vi "UHR-Fleezers Control (host) - 10.7.vi"() -> ()   [LabVIEW 2010] (continued)
    "T2 X" <- w1093
    n789 = Absolute Value(x=w1115) -> (abs(x)=w1116:dbl[])
    n790 = Absolute Value(x=w1114) -> (abs(x)=w1117:dbl[])
    n791 = call <vilib>:"Mean.vi"("X"=w1115) -> ("mean"=w1094:dbl)  [unwired: 1 out]
    "T1 X" <- w1094
    n792 = Add(x=w1116, y=w1117) -> (x+y=w1118:dbl[])
    n793 = Bundle By Name(cluster=w1150, "Y"=w1112) -> (w1080:waveform(dbl))
    "Bead Separation" <- w1080
    n794 = Divide(x=w1118, y=2.0) -> (x/y=→"Vec Mean of T1 T2":dbl[])
    n795 = case shown="True" w1127 {
      tunnel: w1169 -> [_ w2031]
      tunnel: w1168 -> [_ w2030]
      tunnel: w1167 -> [_ w2029]
      tunnel: w1164 -> [_ w2028]
      tunnel: w1089 -> [_ w2027]
      frame False {
      }
      frame True {
        n796 = property on="Force" class="WFChart (strict)"("YScale.NameLbl.Text"=w2031) -> ()  [unwired: 2 in, 2 out]
        n797 = property on="T2 X" class="DigNum (strict)"("Caption.Text"=w2029) -> ()  [unwired: 2 in, 2 out]
        n798 = property on="T1 X" class="DigNum (strict)"("Caption.Text"=w2030) -> ()  [unwired: 2 in, 2 out]
        n799 = property on="Mean" class="DigNum (strict)"("Caption.Text"=w2028) -> ()  [unwired: 2 in, 2 out]
        n800 = property on="Difference" class="DigNum (strict)"("Caption.Text"=w2027) -> ()  [unwired: 2 in, 2 out]
      }
    }
    n801 = local read "Tether"() -> (w1121:bool)
    n802 = Absolute Value(x=w1094) -> (abs(x)=w1091:dbl)
    n803 = Absolute Value(x=w1093) -> (abs(x)=w1090:dbl)
    n804 = Add(x=w1091, y=w1090) -> (x+y=w1166:dbl)
    n805 = Subtract(x=w1091, y=w1090) -> (x-y=→"Difference":dbl)
    n806 = feedback #18(w1112) -> (w1111:dbl[])
    n807 = Divide(x=w1166, y=2.0) -> (x/y=w1120:dbl)
    "Mean" <- w1120
    n808 = case shown="True" w1121 {
      tunnel: w1120 -> [_ w1572]
      frame False {
      }
      frame True {
        n809 = Greater?(x="Lost Tether Alarm Threshold (pN)", y=w1572) -> (0:w1570:bool)
        n810 = case shown="True" w1570 {
          frame False {
          }
          frame True {
            n811 = flat-sequence {
              frame #0 {
                # "stop only if saving"
                n812 = local read "Saving..."() -> (w1585:bool)
                n813 = And(x=w1585, y="TA Cancel Save?") -> (x .and. y?=w1584:bool)
                n814 = local write "Stop Saving"(w1584) -> ()
              }
              frame #1 {
                n815 = case shown="True" "TA Green Off?" {
                  frame False {
                  }
                  frame True {
                    w1588 = FALSE ("Fl. Triggered...")
                    n816 = local write "Fl. Triggered..."(w1588) -> ()
                    n817 = property on="Green Laser ON/Interlacing" class="Bool (strict)"("Val(Sgnl)"=w1588) -> ()  [unwired: 2 in, 2 out]
                  }
                }
              }
            }
            n818 = local read "Time tether formed"() -> (w1579:timestamp)
            n819 = Get Date/Time In Seconds() -> (seconds since 1Jan1904=w1580:timestamp)
            n820 = Subtract(x=w1580, y=w1579) -> (x-y=w1578:dbl)
            n821 = Number To Decimal String(number=w1578) -> (decimal integer string=w1575:string)  [unwired: 1 out]
            n822 = local read "Messages"() -> (w1582:string)
            n823 = call <vilib>:"Beep.vi"() -> ()  [unwired: 3 in, 9 out]
            n824 = Concatenate Strings("Lost tether (" ("Message to add"), w1575, " s)." ("string")) -> (w1577:string)
            n825 = local write "Tether"(FALSE ("Tether")) -> ()
            n826 = call "Update messages.vi"("Message to add"=w1577, "Old message string"=w1582) -> ("New message string"=w1581:string)
            n827 = local write "Messages"(w1581) -> ()
            n828 = property on="Trap Pos. FB ON" class="Bool (strict)"("Val(Sgnl)"=FALSE ("Value (Signaling)")) -> ()  [unwired: 2 in, 2 out]
          }
        }
      }
    }
    n829 = Build Array (concatenate)(w1112, w1111) -> (w1110:dbl[])
    n830 = Split 1D Array(array=w1110, index=w992) -> (first subarray=w1106:dbl[])  [unwired: 1 out]
    n831 = feedback-in #18(w1106) -> ()
    n832 = call <vilib>:"Mean.vi"("X"=w1106) -> ("mean"=w1105:dbl)  [unwired: 1 out]
    "Bead Mean (nm)" <- w1105
    n833 = Subtract(x=w1106, y=w1105) -> (x-y=w1104:dbl[])
    n834 = Square(x=w1104) -> (x^2=w1103:dbl[])
    n835 = call <vilib>:"Mean.vi"("X"=w1103) -> ("mean"=w1102:dbl)  [unwired: 1 out]
    n836 = Square Root(x=w1102) -> (sqrt(x)=w1101:dbl)
    n837 = Multiply(x=10.0, y=w1101) -> (x*y=→"RMS (Ang)":dbl)
    n838 = xnode "Read/Write Control"("FPGA VI Reference In"=w1142, "error in"=w1141) -> ("FPGA VI Reference Out"=w1260:T19, "error out"=w1254:errorcluster, "AI2 Y Sum Set 1"=w1250:i16, "AI2 Y Sum Set 2"=w1249:i16, "AI1 X Set 1"=w1026:fxp<+/-,16,1>, "AI1 X Set 2"=w1025:fxp<+/-,16,1>, "Trap Pos FB Int Signal"=→"Trap Pos FB Int Signal":fxp<+/-,24,9>, "Trap Pos FB Int-Norm Signal"=→"Trap Pos FB Int-Norm Signal":fxp<+/-,16,1>, "Trap Pos FB Action"=w1019:i64, "Scanning"=→"AOD Scanning":bool, "Scan I"=→"AOD Scan I":u64, "Scanning MCL"=w1252:bool, "Scan I (MCL)"=→"MCL Scan I":u64, "Green FB Signals"=w1189:T38)  [unwired: 1 out]
    "MCL Scanning" <- w1252
    "Trap Pos FB Action" <- w1019
    n839 = local read "AI2 (V)"() -> (w1251:cluster{"Set 1":dbl, "Set 2":dbl})
    n840 = Bundle By Name(cluster=w1251, "Set 1"=w1250, "Set 2"=w1249) -> (w1247:cluster{"Set 1":dbl, "Set 2":dbl})
    n841 = Divide(x=w1019, y=327.67) -> (x/y=→"Action (%)":dbl)
    n842 = local read "Trap X (AI1)"() -> (w1039:T10)
    n843 = Divide(x=w1247, y=3276.7) -> (x/y=w1246:cluster{"Set 1":dbl, "Set 2":dbl})
    n844 = local write "AI2 (V)"(w1246) -> ()
    n845 = Bundle(cluster=w1039, "Trap 1"=w1026, "Trap 2"=w1025) -> (→"Trap X (AI1)":T10)
    n846 = Divide(x=w1189, y=3276.7) -> (x/y=w1185:T46)
    n847 = Unbundle By Name(w1185) -> ("Green FB Ch 0"=w1188:dbl, "Green FB Ch 1"=w1187:dbl, "Green FB Ch 2"=w1186:dbl)
    n848 = Divide(x=w1188, y=w1186) -> (x/y=w1184:dbl)
    n849 = Divide(x=w1187, y=w1186) -> (x/y=w1183:dbl)
    n850 = flat-sequence "To save data" {
      tunnel: [w3888] -> w1271
      tunnel: [w3889] -> w1270
      tunnel: w1220 -> [w3882]
      tunnel: w1108 -> [w3886]
      tunnel: ["Save Calibration"] -> w1243
      tunnel: w1240 -> [w3885]
      tunnel: [w3878] -> w1239
      tunnel: [w3875] -> w1238
      tunnel: [w3872] -> w1237
      tunnel: w1219 -> [w3874]
      tunnel: w1125 -> [w3868]
      tunnel: [w3868] -> w1124
      tunnel: ["Start Saving"] -> w1082
      tunnel: [w3862] -> w1008
      tunnel: [w3861] -> w1007
      tunnel: w1271 -> [w4123]
      tunnel: w1270 -> [w4122]
      tunnel: w1009 -> [w4121]
      tunnel: w1243 -> [w4120]
      tunnel: w1239 -> [w4118]
      tunnel: w1238 -> [w4117]
      tunnel: w1237 -> [w4116]
      tunnel: w1095 -> [w4115]
      tunnel: w1134 -> [w4114]
      tunnel: w1124 -> [w4113]
      tunnel: w1082 -> [w4112]
      tunnel: w1080 -> [w4111]
      tunnel: w1056 -> [w4110]
      tunnel: w1008 -> [w4109]
      tunnel: w1007 -> [w4108]
      tunnel: w1006 -> [w4107]
      frame #0 {
        n851 = Or(x="Save N Sets", y="Start Saving") -> (x .or. y?=w3869:bool)
        n852 = To Double Precision Float(number=w3885) -> (double precision float=w3879:dbl)
        n853 = Build Array(w3869, "Save Calibration", w3882, w3874) -> (w3884:bool[])
        n854 = Compound Arithmetic op=OR("Save Calibration", w3882, w3869, w3874) -> (w3887:bool)
        n855 = Boolean Array To Number(Boolean array=w3884) -> (number=w3881:u32)
        n856 = feedback #19(FALSE ("Save APD Data\nwith Trap Data")) -> (w3863:bool)
        n857 = feedback #20(refnum<k0> refnum) -> (w3890:refnum<file>)
        n858 = feedback #21(refnum<k0> refnum) -> (w3865:refnum<file>)
        n859 = feedback #22(FALSE ("Save APD Data\nwith Trap Data")) -> (w3873:bool)
        n860 = feedback #23(refnum<k0> refnum) -> (w3876:refnum<file>)
        n861 = feedback #24(0) -> (w3892:i32)
        n862 = feedback #25() -> (w3880:u32)  [unwired: 1 out]
        n863 = case shown="True" w3887 {
          tunnel: [w3899 1] -> w3888
          tunnel: w3892 -> [w3901 _]
          tunnel: [w3900 w3919] -> w3889
          tunnel: w3890 -> [w3900 _]
          tunnel: w3886 -> [_ w3939]
          tunnel: w3879 -> [_ w3937]
          tunnel: w3881 -> [_ w3940]
          tunnel: [w3898 w3918] -> w3878
          tunnel: w3880 -> [w3898 _]
          tunnel: [w3897 w3916] -> w3875
          tunnel: w3876 -> [w3897 _]
          tunnel: [w3896 w3915] -> w3872
          tunnel: w3873 -> [w3896 _]
          tunnel: "Start Saving" -> [_ w3913]
          tunnel: w3868 -> [_ w3912]
          tunnel: [w3895 w3903] -> w3861
          tunnel: w3865 -> [w3895 _]
          tunnel: [w3894 w3902] -> w3862
          tunnel: w3863 -> [w3894 _]
          frame False {
            n864 = Increment(x=w3901) -> (x+1=w3899:i32)
          }
          frame True {
            w3909 = FALSE ("Start Saving")
            w3914 = 9.0  # File Version
            w3922 = FALSE ("prepend array or string size? (T)")
            w3920 = T39."big-endian, network order" ("byte order (0:big-endian, network order)")
            # "write file headers"
            n865 = local read "BD 1 Frequency 1 (MHz)"() -> (w3936:dbl)
            n866 = local read "BD 2 Frequency 1 (MHz)"() -> (w3935:dbl)
            n867 = local read "BD 1 Frequency 2 (MHz)"() -> (w3934:dbl)
            n868 = local read "BD 2 Frequency 2 (MHz)"() -> (w3933:dbl)
            n869 = local read "BD 1 Frequency 3 (MHz)"() -> (w3932:dbl)
            n870 = local read "BD 2 Frequency 3 (MHz)"() -> (w3931:dbl)
            n871 = Array Size(array=w3912) -> (size(s)=w3911:i32)
            n872 = To Double Precision Float(number=w3911) -> (double precision float=w3910:dbl)
            n873 = local write "Save Calibration"(w3909) -> ()
            n874 = local write "Start Saving"(w3909) -> ()
            n875 = Build Array("Save APD Data\nwith Trap Data", "Save Trap Pos. Data") -> (w3906:bool[])
            n876 = Boolean Array To Number(Boolean array=w3906) -> (number=w3905:u32)
            n877 = Build Array(w3936, w3935, w3934, w3933, w3932, w3931) -> (w3930:dbl[])
            n878 = case shown="2" w3940 {
              tunnel: w3939 -> [w4011 w4031 w4047 w4085]
              tunnel: w3910 -> [w4016 w4038 w4067 w4104]
              tunnel: w3937 -> [w4015 w4037 w4066 w4103]
              tunnel: [w4012 w4033 w4058 w4095] -> w3928
              tunnel: [w4003 "Cal sets to save" w4048 w4086] -> w3918
              tunnel: w3930 -> [w4013 w4034 w4060 w4097]
              tunnel: "Save APD Data\nwith Trap Data" -> [w4010 _ w4044 w4083]
              tunnel: [w4010 w4025 w4044 w4083] -> w3915
              tunnel: w3914 -> [w4006 w4026 w4042 w4081]
              tunnel: w3913 -> [w4005 _ _ _]
              tunnel: [w3996 w4025 w4041 w4071] -> w3902
              tunnel: "Save Trap Pos. Data" -> [w3996 _ w4041 w4071]
              tunnel: w3905 -> [w3995 _ w4040 w4070]
              frame 1, Default {
                # "timeseries"
                n879 = case shown="True" "Profile" {
                  tunnel: [w4019 w4022] -> w4000
                  tunnel: [w4019 w4021] -> w3999
                  tunnel: [w4019 w4020] -> w3998
                  tunnel: [w4019 w4024] -> w3997
                  frame False {
                    w4019 = 0.0 ("f")
                  }
                  frame True {
                    n880 = local read "Current Position"() -> (w4023:dbl[])
                    n881 = local read "Y change (mm)"() -> (w4024:dbl)
                    n882 = call "subVI_explode3array.vi"("Array"=w4023) -> ("x"=w4022:dbl, "y"=w4021:dbl, "z"=w4020:dbl)  [unwired: 12 in]
                  }
                }
                n883 = local read "Save ave N"() -> (w4018:dbl)
                n884 = Multiply(x=w4018, y=w4011) -> (x*y=w4017:dbl)
                n885 = To Double Precision Float(number=w3995) -> (double precision float=w4009:dbl)
                n886 = Build Array(w4006, w4011, w4017, w4016, w4015, 0.0 ("f")) -> (w4014:dbl[])
                n887 = Build Array(w4009, w4000, w3999, w3998, w3997) -> (w4007:dbl[])
                n888 = Select(t=u32 4000000000, s=w4005, f="N sets to save") -> (s? t:f=w4003:u32)
                n889 = Build Array (concatenate)(w4014, w4013, w4007) -> (w4012:dbl[])
              }
              frame 2 {
                w4028 = 0.0 ("f")
                w4025 = FALSE ("Save APD Data\nwith Trap Data")
                # "calibration"
                n890 = Boolean To (0,1)(Boolean=w4025) -> (0, 1=w4030:i16)
                n891 = To Double Precision Float(number=w4030) -> (double precision float=w4029:dbl)
                n892 = Build Array(w4029, w4028, w4028, w4028, w4028) -> (w4027:dbl[])
                n893 = Build Array(w4026, w4031, w4031, w4038, w4037, 1.0 ("t")) -> (w4035:dbl[])
                n894 = Build Array (concatenate)(w4035, w4034, w4027) -> (w4033:dbl[])
                "Calibrating Trap..." <- TRUE ("Calibrating...")
              }
              frame 4 {
                w4045 = 0.0 ("f")
                # "scan dir (x/y = 0/1)"
                # "cycles/step"
                # "n scans (f/b)"
                # "steps"
                # "freq. range"
                # "AOD raster scan"
                n895 = local read "Number of F/B Scans (AOD)"() -> (w4052:u16)
                n896 = local read "Cycles/step (AOD)"() -> (w4054:u64)
                n897 = local read "Scan Range (MHz)"() -> (w4057:dbl)
                n898 = local read "Scan steps (AOD)"() -> (w4056:u64)
                n899 = local read "Scan BD"() -> (w4064:bool)
                n900 = local read "Save ave N"() -> (w4069:dbl)
                n901 = Boolean To (0,1)(Boolean=w4064) -> (0, 1=w4063:i16)
                n902 = To Double Precision Float(number=w4052) -> (double precision float=w4051:dbl)
                n903 = To Double Precision Float(number=w4056) -> (double precision float=w4055:dbl)
                n904 = To Double Precision Float(number=w4054) -> (double precision float=w4053:dbl)
                n905 = To Double Precision Float(number=w4063) -> (double precision float=w4062:dbl)
                n906 = Multiply(x=w4069, y=w4047) -> (x*y=w4068:dbl)
                n907 = To Double Precision Float(number=w4040) -> (double precision float=w4046:dbl)
                n908 = Build Array(w4046, w4045, w4045, w4045, w4045) -> (w4043:dbl[])
                n909 = local read "N sets should be saved"() -> (w4049:dbl)
                n910 = Build Array(w4062, w4057, w4055, w4053, w4051) -> (w4059:dbl[])
                n911 = Build Array(w4042, w4047, w4068, w4067, w4066, 2.0 ("t")) -> (w4061:dbl[])
                n912 = Round Toward +Infinity(x=w4049) -> (ceil(x): smallest int >= x=w4050:dbl)
                n913 = Build Array (concatenate)(w4061, w4060, w4043, w4059) -> (w4058:dbl[])
                n914 = To Unsigned Long Integer(number=w4050) -> (unsigned 32bit integer=w4048:u32)
              }
              frame 8 {
                w4078 = 0.0 ("f")
                # "MCL raster scan"
                n915 = local read "Number of scans (MCL)"() -> (w4073:u64)
                n916 = local read "Scan lines (y)"() -> (w4072:u64)
                n917 = local read "2D or 1D Scan"() -> (w4075:bool)
                n918 = local read "Scan Range (V)\n(of steps)"() -> (w4094:dbl)
                n919 = local read "Fast Scan Dir"() -> (w4101:bool)
                n920 = local read "Cycles/step (MCL)"() -> (w4091:u64)
                n921 = local read "Scan steps (MCL)"() -> (w4093:u64)
                n922 = Select(t=w4072, s=w4075, f=w4073) -> (s? t:f=w4074:u64)
                n923 = Boolean To (0,1)(Boolean=w4075) -> (0, 1=w4077:i16)
                n924 = local read "Save ave N"() -> (w4106:dbl)
                n925 = local read "Initial X"() -> (w4080:dbl)
                n926 = local read "Initial Y"() -> (w4079:dbl)
                n927 = To Double Precision Float(number=w4077) -> (double precision float=w4076:dbl)
                n928 = Boolean To (0,1)(Boolean=w4101) -> (0, 1=w4100:i16)
                n929 = To Double Precision Float(number=w4074) -> (double precision float=w4089:dbl)
                n930 = To Double Precision Float(number=w4093) -> (double precision float=w4092:dbl)
                n931 = To Double Precision Float(number=w4091) -> (double precision float=w4090:dbl)
                n932 = To Double Precision Float(number=w4100) -> (double precision float=w4099:dbl)
                n933 = Multiply(x=w4106, y=w4085) -> (x*y=w4105:dbl)
                n934 = To Double Precision Float(number=w4070) -> (double precision float=w4084:dbl)
                n935 = local read "N sets should be saved (MCL)"() -> (w4087:dbl)
                n936 = Build Array(w4084, w4076, w4078, w4078, w4078) -> (w4082:dbl[])
                n937 = Build Array(w4099, w4094, w4092, w4090, w4089, w4080, w4079) -> (w4096:dbl[])
                n938 = Build Array(w4081, w4085, w4105, w4104, w4103, 3.0 ("t")) -> (w4098:dbl[])
                n939 = Round Toward +Infinity(x=w4087) -> (ceil(x): smallest int >= x=w4088:dbl)
                n940 = Build Array (concatenate)(w4098, w4097, w4082, w4096) -> (w4095:dbl[])
                n941 = To Unsigned Long Integer(number=w4088) -> (unsigned 32bit integer=w4086:u32)
              }
            }
            n942 = local read "Index"() -> (w3945:dbl)
            n943 = call "Create new save file.vi"("Insert"="", "Ext"=".dat", "Index In"=w3945) -> ("Path Out"=w3904:path, "Index Out"=w3917:dbl)
            n944 = local write "Save file name"(w3904) -> ()
            n945 = local write "Index"(w3917) -> ()
            n946 = local write "Save index"(w3917) -> ()
            n947 = Array Size(array=w3928) -> (size(s)=w3929:i32)
            n948 = Open/Create/Replace File(file path (use dialog)=w3904, operation (0:open)=T25."create", access (0:read/write)=enum16{"read/write", "read-only", "write-only"}."write-only") -> (refnum out=w3942:refnum<file>)  [unwired: 1 in, 4 out]
            n949 = local write "Saving..."(TRUE ("Saving...")) -> ()
            n950 = To Double Precision Float(number=w3929) -> (double precision float=w3927:dbl)
            n951 = String Length(string="Comment (data description)") -> (length=w3925:i32)
            n952 = To Double Precision Float(number=w3925) -> (double precision float=w3924:dbl)
            n953 = Deny Access(7:w3942) -> (3:w3941:refnum<file>)  [unwired: 1 in, 2 out]
            n954 = Build Array (concatenate)(w3927, w3928, w3924) -> (w3926:dbl[])
            n955 = case "If fluorescence data to be saved" shown="False" w3915 {
              tunnel: w3904 -> [_ w3994]
              tunnel: [refnum<k0> refnum w3974] -> w3916
              frame False {
              }
              frame True {
                w3973 = 0.0
                n956 = local read "APD Integration Time (s)"() -> (w3979:dbl)
                n957 = local read "N APD Samp/step"() -> (w3972:dbl)
                n958 = Path To String(path=w3994) -> (string=w3993:string)
                n959 = String Length(string=w3993) -> (length=w3992:i32)
                n960 = Subtract(x=w3992, y=4) -> (x-y=w3990:i32)
                n961 = String Subset(string=w3993, length (rest)=w3990) -> (substring=w3989:string)  [unwired: 1 out]
                n962 = Build Array(w3979, w3972, w3973, w3973, w3973, w3973, w3973, w3973) -> (w3976:dbl[])
                n963 = Concatenate Strings(w3989, "_fl.dat" ("string")) -> (w3987:string)
                n964 = Array Size(array=w3976) -> (size(s)=w3978:i32)
                n965 = String To Path(string=w3987) -> (path=w3983:path)
                n966 = Open/Create/Replace File(file path (use dialog)=w3983, operation (0:open)=T25."create", access (0:read/write)=enum16{"read/write", "read-only", "write-only"}."write-only") -> (refnum out=w3984:refnum<file>)  [unwired: 1 in, 4 out]
                n967 = Deny Access(7:w3984) -> (3:w3980:refnum<file>)  [unwired: 1 in, 2 out]
                n968 = To Double Precision Float(number=w3978) -> (double precision float=w3977:dbl)
                n969 = Build Array (concatenate)(w3977, w3976) -> (w3975:dbl[])
                n970 = Write to Binary File(file (use dialog)=w3980, data=w3975, 5:FALSE ("prepend array or string size? (T)"), 9:T39."big-endian, network order" ("byte order (0:big-endian, network order)")) -> (refnum out=w3974:refnum<file>)  [unwired: 1 in, 3 out]
              }
            }
            n971 = case shown="False" w3902 {
              tunnel: w3904 -> [_ w3956]
              tunnel: [refnum<k0> refnum w3955] -> w3903
              frame False {
              }
              frame True {
                w3951 = 0.0 ("element")
                n972 = Path To String(path=w3956) -> (string=w3970:string)
                n973 = Build Array(w3951, w3951, w3951, w3951, w3951, w3951, w3951, w3951) -> (w3952:dbl[])
                n974 = String Length(string=w3970) -> (length=w3969:i32)
                n975 = Subtract(x=w3969, y=4) -> (x-y=w3967:i32)
                n976 = Array Size(array=w3952) -> (size(s)=w3954:i32)
                n977 = String Subset(string=w3970, length (rest)=w3967) -> (substring=w3966:string)  [unwired: 1 out]
                n978 = To Double Precision Float(number=w3954) -> (double precision float=w3953:dbl)
                n979 = Concatenate Strings(w3966, "_pos.dat" ("string")) -> (w3964:string)
                n980 = Build Array (concatenate)(w3953, w3952) -> (w3950:dbl[])
                n981 = String To Path(string=w3964) -> (path=w3960:path)
                n982 = Open/Create/Replace File(file path (use dialog)=w3960, operation (0:open)=T25."create", access (0:read/write)=enum16{"read/write", "read-only", "write-only"}."write-only") -> (refnum out=w3961:refnum<file>)  [unwired: 1 in, 4 out]
                n983 = Deny Access(7:w3961) -> (3:w3957:refnum<file>)  [unwired: 1 in, 2 out]
                n984 = Write to Binary File(file (use dialog)=w3957, data=w3950, 5:FALSE ("prepend array or string size? (T)"), 9:T39."big-endian, network order" ("byte order (0:big-endian, network order)")) -> (refnum out=w3955:refnum<file>)  [unwired: 1 in, 3 out]
              }
            }
            n985 = Write to Binary File(file (use dialog)=w3941, data=w3926, 5:w3922, 9:w3920) -> (refnum out=w3923:refnum<file>)  [unwired: 1 in, 3 out]
            n986 = Write to Binary File(file (use dialog)=w3923, data="Comment (data description)", 5:w3922, 9:w3920) -> (refnum out=w3919:refnum<file>)  [unwired: 1 in, 3 out]
          }
        }
        n987 = feedback-in #19(w3862) -> ()
        n988 = feedback-in #20(w3889) -> ()
        n989 = feedback-in #21(w3861) -> ()
        n990 = feedback-in #22(w3872) -> ()
        n991 = feedback-in #23(w3875) -> ()
        n992 = feedback-in #24(w3888) -> ()
        n993 = feedback-in #25(w3878) -> ()
      }
      frame #1 {
        n994 = local read "Saving..."() -> (w4119:bool)
        n995 = case shown="True" w4119 {
          tunnel: w4123 -> [_ w4133]
          tunnel: w4122 -> [_ w4147]
          tunnel: w4121 -> [_ w4143]
          tunnel: w4120 -> [_ w4142]
          tunnel: w4118 -> [_ w4141]
          tunnel: w4117 -> [_ w4136]
          tunnel: w4116 -> [_ w4135]
          tunnel: w4115 -> [_ w4134]
          tunnel: w4114 -> [_ w4132]
          tunnel: w4113 -> [_ w4130]
          tunnel: w4112 -> [_ w4129]
          tunnel: w4111 -> [_ w4128]
          tunnel: w4110 -> [_ w4127]
          tunnel: w4109 -> [_ w4126]
          tunnel: w4108 -> [_ w4125]
          tunnel: w4107 -> [_ w4124]
          frame False {
          }
          frame True {
            n996 = Multiply(x=w4133, y=w4132) -> (x*y=→"Time (s)":dbl)
            n997 = Less Or Equal?(x=w4133, y=w4141) -> (x <= y?=w4145:bool)
            n998 = Or(x="Stop Saving", y="Abort save 2") -> (x .or. y?=w4137:bool)
            n999 = Not(x=w4137) -> (.not. x?=w4146:bool)
            n1000 = And(x=w4145, y=w4146) -> (x .and. y?=w4144:bool)
            n1001 = case shown="False" w4144 {
              tunnel: w4147 -> [w4154 w4222]
              tunnel: [0.0 w4225] -> w4140
              tunnel: w4133 -> [_ w4223]
              tunnel: w4141 -> [_ w4224]
              tunnel: w4143 -> [_ w4219]
              tunnel: w4142 -> [_ _]
              tunnel: w4136 -> [w4152 w4212]
              tunnel: w4135 -> [w4151 w4213]
              tunnel: w4134 -> [_ w4211]
              tunnel: w4130 -> [_ w4210]
              tunnel: w4129 -> [_ w4164]
              tunnel: w4128 -> [_ w4203]
              tunnel: w4127 -> [_ w4181]
              tunnel: w4126 -> [w4148 w4162]
              tunnel: w4125 -> [w4149 w4161]
              tunnel: w4124 -> [_ w4158]
              frame False {
                w4150 = FALSE
                n1002 = Close File(refnum=w4154) -> ()  [unwired: 1 in, 2 out]
                n1003 = case shown="True" w4151 {
                  tunnel: w4152 -> [_ w4156]
                  frame False {
                  }
                  frame True {
                    n1004 = Close File(refnum=w4156) -> ()  [unwired: 1 in, 2 out]
                  }
                }
                n1005 = case shown="True" w4148 {
                  tunnel: w4149 -> [_ w4155]
                  frame False {
                  }
                  frame True {
                    n1006 = Close File(refnum=w4155) -> ()  [unwired: 1 in, 2 out]
                  }
                }
                n1007 = local write "Raster Scanning..."(w4150) -> ()
                n1008 = local write "Calibrating Trap..."(w4150) -> ()
                n1009 = call <vilib>:"Beep.vi"() -> ()  [unwired: 3 in, 9 out]
                n1010 = local write "Stop Saving"(w4150) -> ()
                "Saving..." <- w4150
              }
              frame True {
                n1011 = local read "Calibrating Trap..."() -> (w4214:bool)
                n1012 = case "Write fl. data" shown="False" w4213 {
                  tunnel: w4212 -> [_ w4248]
                  tunnel: w4211 -> [_ w4247]
                  frame False {
                  }
                  frame True {
                    n1013 = Write to Binary File(file (use dialog)=w4248, data=w4247, 5:FALSE ("prepend array or string size? (T)"), 9:T39."big-endian, network order" ("byte order (0:big-endian, network order)")) -> ()  [unwired: 1 in, 4 out]
                  }
                }
                n1014 = Greater?(x="Save ave N", y=1.0) -> (0:w4217:bool)
                n1015 = Not(x=w4214) -> (.not. x?=w4216:bool)
                n1016 = And(x=w4216, y=w4217) -> (x .and. y?=w4159:bool)
                n1017 = case shown="True" w4159 {
                  tunnel: w4158 -> [w4228 w4239]
                  tunnel: [w4228 w4231] -> w4157
                  tunnel: "Save ave N" -> [_ w4232]
                  frame False {
                  }
                  frame True {
                    w4229 = 2 ("dimension size")
                    n1018 = Array Size(array=w4239) -> (size(s)=w4233:i32)
                    n1019 = Divide(x=w4233, y=w4229) -> (x/y=w4237:dbl)
                    n1020 = Reshape Array(w4239, w4237, w4229) -> (w4238:u64[][])
                    n1021 = Transpose 2D Array(2D array=w4238) -> (transposed array=w4236:u64[][])
                    n1022 = for {
                      tunnel: w4236 -> [w4241] mode=indexing
                      tunnel: [w4240] -> w4230 mode=indexing
                      tunnel: w4232 -> [w4242]
                      workers-P: _ -> [_]
                      n1023 = call "downsample 1D array - U64.vi"("Ave N"=w4242, "Array In"=w4241) -> ("Array Out"=w4240:u64[])  [unwired: 1 in]
                    }
                    n1024 = Transpose 2D Array(2D array=w4230) -> (transposed array=w4235:u64[][])
                    n1025 = Divide(x=w4233, y=w4232) -> (x/y=w4234:dbl)
                    n1026 = Reshape Array(w4235, w4234) -> (w4231:u64[])
                  }
                }
                n1027 = case shown="False" w4159 {
                  tunnel: w4219 -> [w4251 w4263]
                  tunnel: [w4251 w4255] -> w4215
                  tunnel: "Save ave N" -> [_ w4256]
                  tunnel: w4210 -> [_ w4254]
                  frame False {
                    # "don't downsample data for trap calibration"
                  }
                  frame True {
                    n1028 = Array Size(array=w4263) -> (size(s)=w4257:i32)
                    n1029 = Array Size(array=w4254) -> (size(s)=w4253:i32)
                    n1030 = Divide(x=w4257, y=w4253) -> (x/y=w4261:dbl)
                    n1031 = Reshape Array(w4263, w4261, w4253) -> (w4262:i16[][])
                    n1032 = Transpose 2D Array(2D array=w4262) -> (transposed array=w4260:i16[][])
                    n1033 = for {
                      tunnel: w4260 -> [w4266] mode=indexing
                      tunnel: [w4265] -> w4252 mode=indexing
                      tunnel: w4256 -> [w4264]
                      workers-P: _ -> [_]
                      n1034 = call "downsample 1D array - I16.vi"("Ave N"=w4264, "Array In"=w4266) -> ("Array Out"=w4265:i16[])  [unwired: 1 out]
                    }
                    n1035 = Transpose 2D Array(2D array=w4252) -> (transposed array=w4259:i16[][])
                    n1036 = Divide(x=w4257, y=w4256) -> (x/y=w4258:dbl)
                    n1037 = Reshape Array(w4259, w4258) -> (w4255:i16[])
                  }
                }
                n1038 = Index Array(array=w4181, index=1) -> (element=w4184:waveform(dbl))
                n1039 = Index Array(array=w4181, index=0) -> (element=w4186:waveform(dbl))
                n1040 = Unbundle By Name(w4184) -> ("Y"=w4188:dbl[])
                n1041 = Unbundle By Name(w4186) -> ("Y"=w4196:dbl[])
                n1042 = case "Write trap pos. data" shown="True" w4162 {
                  tunnel: w4161 -> [_ w4244]
                  tunnel: w4157 -> [_ w4243]
                  frame False {
                  }
                  frame True {
                    n1043 = Write to Binary File(file (use dialog)=w4244, data=w4243, 5:FALSE ("prepend array or string size? (T)"), 9:T39."big-endian, network order" ("byte order (0:big-endian, network order)")) -> ()  [unwired: 1 in, 4 out]
                  }
                }
                n1044 = Write to Binary File(file (use dialog)=w4222, data=w4215, 5:FALSE ("prepend array or string size? (T)"), 9:T39."big-endian, network order" ("byte order (0:big-endian, network order)")) -> ()  [unwired: 1 in, 4 out]
                n1045 = feedback #26(w4188) -> (w4190:dbl[])
                n1046 = Build Array (concatenate)(w4190, w4188) -> (w4189:dbl[])
                n1047 = Select(t=w4188, s=w4164, f=w4189) -> (s? t:f=w4174:dbl[])
                n1048 = feedback-in #26(w4174) -> ()
                n1049 = feedback #27(w4196) -> (w4209:dbl[])
                n1050 = Build Array (concatenate)(w4209, w4196) -> (w4208:dbl[])
                n1051 = Select(t=w4196, s=w4164, f=w4208) -> (s? t:f=w4183:dbl[])
                n1052 = feedback-in #27(w4183) -> ()
                n1053 = Divide(x=w4223, y=w4224) -> (x/y=w4226:dbl)
                n1054 = Multiply(x=w4226, y=100.0) -> (x*y=w4225:dbl)
                n1055 = Build Array(w4183, w4174) -> (→"Saved APD":dbl[][])
                n1056 = Array Size(array=w4183) -> (size(s)=w4201:i32)
                n1057 = Unbundle By Name(w4203) -> ("Y"=w4207:dbl[])
                n1058 = Subtract(x=w4201, y="N pts to average") -> (x-y=w4177:i32)
                n1059 = Multiply(x="N pts to average", y=u16 2) -> (x*y=w4178:u16)
                n1060 = Subtract(x=w4201, y=w4178) -> (x-y=w4176:i32)
                n1061 = feedback #28(w4207) -> (w4206:dbl[])
                n1062 = Build Array (concatenate)(w4206, w4207) -> (w4205:dbl[])
                n1063 = Select(t=w4207, s=w4164, f=w4205) -> (s? t:f=w4204:dbl[])
                "Trap Delta Graph" <- w4204
                n1064 = feedback-in #28(w4204) -> ()
                n1065 = Array Subset(array=w4183, index=w4177, length="N pts to average") -> (w4200:dbl[])
                n1066 = Array Subset(array=w4183, index=w4176, length="N pts to average") -> (w4199:dbl[])
                n1067 = Array Subset(array=w4174, index=w4177, length="N pts to average") -> (w4180:dbl[])
                n1068 = Array Subset(array=w4174, index=w4176, length="N pts to average") -> (w4179:dbl[])
                n1069 = call <vilib>:"Mean.vi"("X"=w4200) -> ("mean"=w4198:dbl)  [unwired: 1 out]
                n1070 = call <vilib>:"Mean.vi"("X"=w4180) -> ("mean"=w4173:dbl)  [unwired: 1 out]
                n1071 = call <vilib>:"Mean.vi"("X"=w4199) -> ("mean"=w4197:dbl)  [unwired: 1 out]
                n1072 = call <vilib>:"Mean.vi"("X"=w4179) -> ("mean"=w4172:dbl)  [unwired: 1 out]
                n1073 = Subtract(x=w4173, y=w4172) -> (x-y=w4163:dbl)
                "Delta Fl. 2" <- w4163
                n1074 = Subtract(x=w4198, y=w4197) -> (x-y=w4195:dbl)
                "Delta Fl. 1" <- w4195
                n1075 = Initialize Array(w4195, 1 ("dimension size")) -> (w4192:dbl[])
                n1076 = Initialize Array(w4163, 1 ("dimension size")) -> (w4169:dbl[])
                n1077 = feedback #29(w4192) -> (w4193:dbl[])
                n1078 = Build Array (concatenate)(w4193, w4192) -> (w4191:dbl[])
                n1079 = feedback #30(w4169) -> (w4170:dbl[])
                n1080 = Build Array (concatenate)(w4170, w4169) -> (w4168:dbl[])
                n1081 = Select(t=w4192, s=w4164, f=w4191) -> (s? t:f=w4167:dbl[])
                n1082 = feedback-in #29(w4167) -> ()
                n1083 = Select(t=w4169, s=w4164, f=w4168) -> (s? t:f=w4166:dbl[])
                n1084 = feedback-in #30(w4166) -> ()
                n1085 = Build Array(w4167, w4166) -> (→"Save APD Deriv":dbl[][])
              }
            }
            "Progress" <- w4140
            "Progress 2" <- w4140
          }
        }
      }
    }
    n1086 = Bundle By Name(cluster=w1185, "Green FB Ch 0"=w1184, "Green FB Ch 1"=w1183) -> (w1163:T46)
    "Green FB Signals (V)" <- w1163
    n1087 = Unbundle By Name(w1163) -> ("Green FB Ch 2"=→"Green FB Plot":dbl)
    n1088 = local read "wait to reset values"() -> (w1255:bool)
    n1089 = Not(x=w1252) -> (.not. x?=w1256:bool)
    n1090 = And(x=w1256, y=w1255) -> (x .and. y?=w1257:bool)
    n1091 = case "Part of MCL raster scanning: returns to initial positions after scan done" shown="True" w1257 {
      tunnel: w1260 -> [w2857 w2864]
      tunnel: [w2857 w2863] -> w1259
      tunnel: w1254 -> [w2856 w2862]
      tunnel: [w2856 w2861] -> w1253
      frame False {
      }
      frame True {
        w2872 = 10.0 ("y")
        w2871 = 32767.0 ("y")
        # "to return scan values\nafter a synchronous \nAOM scan"
        n1092 = local read "AO2"() -> (w2865:dbl)
        n1093 = local read "AO1"() -> (w2866:dbl)
        n1094 = local write "wait to reset values"(FALSE ("wait to reset values")) -> ()
        n1095 = Multiply(x=w2866, y=w2871) -> (x*y=w2868:dbl)
        n1096 = Multiply(x=w2865, y=w2871) -> (x*y=w2870:dbl)
        n1097 = Divide(x=w2868, y=w2872) -> (x/y=w2867:dbl)
        n1098 = Divide(x=w2870, y=w2872) -> (x/y=w2869:dbl)
        n1099 = To Word Integer(number=w2867) -> (16bit integer=w2873:i16)
        n1100 = To Word Integer(number=w2869) -> (16bit integer=w2874:i16)
        n1101 = local read "Total Counts (ticks)"() -> (w2858:u32)
        n1102 = xnode "Read/Write Control"("FPGA VI Reference In"=w2864, "error in"=w2862, "AO1"=w2873, "AO2"=w2874, "MCL count"=w2858) -> ("FPGA VI Reference Out"=w2863:T19, "error out"=w2861:errorcluster)
        n1103 = local read "Scan Range (V)\n(of steps)"() -> (w2859:dbl)
        n1104 = property on="Scan Range (V)\n(of steps)" class="DigNum (strict)"("Val(Sgnl)"=w2859) -> ()  [unwired: 2 in, 2 out]
      }
    }
    n1105 = node-c288() -> ()  [unwired: 2 out]
  }
  n1106 = node-c288(3 ("Processor")) -> (w73:T26)  [unwired: 3 out]
  n1107 = disable-structure shown="Enabled" {
    disable-tunnel: [w4268 _] -> w32
    disable-tunnel: w16 -> [w4267 _]
    frame Enabled {
      n1108 = node-c288() -> (w4270:T26)  [unwired: 4 out]
      n1109 = timed-loop "Rough control of MCL mirror stage (debugging)" {
        tunnel: w4267 -> [w4273]
        tunnel: [w4272] -> w4268
        timing: w4270 -> [_]
        timing-out: [_] -> w4269
        stop <- w4272 stop-if-true
        n1110 = node-c288() -> ()  [unwired: 2 out]
        n1111 = case shown="1" "MCL Mode" {
          tunnel: w4273 -> [_ w4276 w4380]
          frame 0, Default {
            # "manual positioning"
          }
          frame 1 {
            # "sinusoidal wave"
            n1112 = node-c288() -> (w4278:T26)  [unwired: 4 out]
            n1113 = timed-loop "Oscillate MCL mirror" {
              timing: w4278 -> [_]
              timing-out: [_] -> w4277
              tunnel: w4276 -> [w4317]
              i -> [w4316]
              stop <- w4279 stop-if-true
              n1114 = node-c288() -> (w4315:i64)  [unwired: 1 out]
              n1115 = Multiply(x="AO1", y=32767.0) -> (x*y=w4311:dbl)
              n1116 = Multiply(x="AO2", y=32767.0) -> (x*y=w4306:dbl)
              n1117 = Divide(x=w4311, y=10.0) -> (x/y=w4312:dbl)
              n1118 = Divide(x=w4306, y=10.0) -> (x/y=w4307:dbl)
              n1119 = To Word Integer(number=w4312) -> (16bit integer=w4304:i16)
              n1120 = To Word Integer(number=w4307) -> (16bit integer=w4303:i16)
              n1121 = Divide(x=w4315, y=i64 1000) -> (x/y=w4286:dbl)
              n1122 = Multiply(x=w4286, y=w4316) -> (x*y=w4297:dbl)
              n1123 = Multiply(x="Osc. freq. (Hz) 2", y=6.283185307179586) -> (x*y=w4298:dbl)
              n1124 = Multiply(x=w4298, y=w4297) -> (x*y=w4296:dbl)
              n1125 = Sine(x=w4296) -> (sin(x)=w4295:dbl)
              n1126 = Multiply(x=w4295, y="Osc. amp. (V)") -> (x*y=w4293:dbl)
              n1127 = Add(x=w4293, y="Osc. center (V)") -> (x+y=w4291:dbl)
              n1128 = Divide(x=w4291, y=10.0) -> (x/y=w4289:dbl)
              n1129 = Multiply(x=w4289, y=32767.0) -> (x*y=w4284:dbl)
              n1130 = Select(t=w4284, s="Scan axis", f=w4304) -> (s? t:f=w4302:dbl)
              n1131 = Select(t=w4303, s="Scan axis", f=w4284) -> (s? t:f=w4301:dbl)
              n1132 = local read "MCL Mode"() -> (w4283:u16)
              n1133 = Not Equal?(x=w4283, y=u16 1) -> (x != y?=w4280:bool)
              n1134 = local read "Stop All"() -> (w4281:bool)
              n1135 = xnode "Read/Write Control"("FPGA VI Reference In"=w4317, "AO1"=w4302, "AO2"=w4301) -> ()  [unwired: 1 in, 2 out]
              n1136 = Compound Arithmetic op=OR(w4281, w4280) -> (w4279:bool)
              n1137 = node-c288() -> ()  [unwired: 2 out]
            }
            n1138 = node-c288(w4277) -> ()  [unwired: 1 out]
          }
          frame 2 {
            # "linear scan"
            n1139 = case shown="True" "Start Scan" {
              tunnel: w4380 -> [_ w4392]
              frame False {
              }
              frame True {
                n1140 = Subtract(x="End (V)", y="Begin (V)") -> (x-y=w4388:dbl)
                n1141 = Decrement(x="N Points") -> (x-1=w4387:dbl)
                n1142 = Divide(x=w4388, y=w4387) -> (x/y=w4385:dbl)
                n1143 = for {
                  N: "N Points" -> [_]
                  tunnel: "Begin (V)" -> [w4405]
                  tunnel: w4392 -> [w4397]
                  tunnel: [w4396] -> w4391 mode=indexing
                  tunnel: w4385 -> [w4395]
                  tunnel: [w4393] -> w4384 mode=indexing
                  i -> [w4404]
                  n1144 = Multiply(x=w4395, y=w4404) -> (x*y=w4403:dbl)
                  n1145 = Add(x=w4405, y=w4403) -> (x+y=w4400:dbl)
                  n1146 = local read "Scan axis"() -> (w4394:bool)
                  n1147 = local read "AO1"() -> (w4402:dbl)
                  n1148 = local read "AO2"() -> (w4401:dbl)
                  n1149 = Select(t=w4400, s=w4394, f=w4402) -> (s? t:f=w4399:dbl)
                  n1150 = Select(t=w4401, s=w4394, f=w4400) -> (s? t:f=w4398:dbl)
                  n1151 = flat-sequence {
                    tunnel: w4399 -> [w4409]
                    tunnel: w4398 -> [w4408]
                    tunnel: w4397 -> [w4406]
                    tunnel: [w4476] -> w4396
                    tunnel: [w4475] -> w4393
                    frame #0 {
                      w4412 = 10.0 ("y")
                      w4407 = 32767.0 ("y")
                      n1152 = Multiply(x=w4409, y=w4407) -> (x*y=w4415:dbl)
                      n1153 = Multiply(x=w4408, y=w4407) -> (x*y=w4413:dbl)
                      n1154 = Divide(x=w4415, y=w4412) -> (x/y=w4416:dbl)
                      n1155 = Divide(x=w4413, y=w4412) -> (x/y=w4414:dbl)
                      n1156 = To Word Integer(number=w4416) -> (16bit integer=w4410:i16)
                      n1157 = To Word Integer(number=w4414) -> (16bit integer=w4411:i16)
                      n1158 = xnode "Read/Write Control"("FPGA VI Reference In"=w4406, "AO1"=w4410, "AO2"=w4411) -> ()  [unwired: 1 in, 2 out]
                    }
                    frame #1 {
                      n1159 = Wait (ms)(milliseconds to wait="DAQ Delay (ms)") -> ()  [unwired: 1 out]
                    }
                    frame #2 {
                      n1160 = local read "Slow mean"() -> (w4476:dbl)
                      n1161 = local read "Sigma"() -> (w4475:dbl)
                    }
                  }
                }
                n1162 = Bundle("Begin (V)"="Begin (V)", w4385, w4391) -> (→"MCL Scan":cluster{"Begin (V)":dbl, dbl, dbl[]})  [unwired: 1 out]
                n1163 = Bundle("Begin (V)"="Begin (V)", w4385, w4384) -> (→"MCL Scan 2":cluster{"Begin (V)":dbl, dbl, dbl[]})  [unwired: 1 out]
              }
            }
          }
        }
        n1164 = local read "Stop All"() -> (w4272:bool)
        n1165 = node-c288() -> ()  [unwired: 2 out]
      }
      n1166 = node-c288(w4269) -> ()  [unwired: 1 out]
    }
    frame Disabled {
    }
  }
  n1167 = timed-loop "Control parameters (event loop)" {
    tunnel: w16 -> [w4482]
    shift-right: [w4481] -> _
    shift-left: errorcluster {"status"=FALSE, "code"=0, "source"=""} ("error out") -> [w4480]
    tunnel: [w4479] -> w34
    timing: w7 -> [_]
    timing-out: [_] -> w6
    stop <- w4479 stop-if-true
    n1168 = node-c288() -> ()  [unwired: 1 in, 1 out]
    n1169 = event shown="[44] \"Inject Top\": Value Change" {
      selector: _ -> [_ _ _ _ _ _ _ _ _ _ _ _ _ _ _ _ _ _ _ _ _ _ _ _ _ _ _ _ _ _ _ _ _ _ _ _ _ _ _ _ _ _ _ _ _ _ _ _ _ _ _ _ _ _ _ _]
      dyn-events: _ -> [_ _ _ _ _ _ _ _ _ _ _ _ _ _ _ _ _ _ _ _ _ _ _ _ _ _ _ _ _ _ _ _ _ _ _ _ _ _ _ _ _ _ _ _ _ _ _ _ _ _ _ _ _ _ _ _]
      timeout: _ -> [_ _ _ _ _ _ _ _ _ _ _ _ _ _ _ _ _ _ _ _ _ _ _ _ _ _ _ _ _ _ _ _ _ _ _ _ _ _ _ _ _ _ _ _ _ _ _ _ _ _ _ _ _ _ _ _]
      tunnel: w4482 -> [w4520 _ _ _ w4642 _ w4739 _ w4803 _ _ _ w4998 _ _ w5100 w5244 w5308 w5383 w5537 w5614 w5745 _ w5841 w5927 w6013 w6099 w6185 w6271 w6364 w6528 w6739 w6882 w7019 _ _ w7287 w7329 w7377 w7456 w7498 _ w7544 _ _ _ _ w7735 _ w7828 w7869 w7916 w8104 w8153 _ w8215]
      tunnel: [w4519 _ _ _ w4632 _ w4738 _ w4766 _ w4963 _ w4977 _ _ w5099 w5240 w5305 w5380 w5536 w5612 w5744 _ w5835 w5921 w6007 w6093 w6179 w6265 w6362 w6527 w6737 w6880 w7017 _ _ w7285 w7327 w7367 w7454 w7496 _ w7542 _ _ _ _ w7733 _ _ _ _ _ _ _ _] -> w4481
      tunnel: w4480 -> [w4518 _ _ _ w4641 _ w4737 _ w4798 _ w4963 _ w4997 _ _ w5098 w5239 w5304 w5379 w5535 w5613 w5743 _ w5840 w5926 w6012 w6098 w6184 w6270 w6363 w6526 w6738 w6881 w7018 _ _ w7286 w7328 w7376 w7455 w7497 _ w7543 _ _ _ _ w7734 _ w7827 w7868 w7915 w8103 w8152 _ w8214]
      tunnel: [_ _ _ _ _ _ _ _ _ _ w4962 _ _ _ _ _ _ _ _ _ _ _ _ _ _ _ _ _ _ _ _ _ _ _ _ _ _ _ _ _ _ _ _ _ _ _ _ _ _ _ _ _ _ _ _ _] -> w4479
      tunnel: [_ _ _ _ _ _ _ "Round T1 X" _ _ _ _ _ _ _ _ _ _ _ _ _ _ _ _ _ _ _ _ _ _ _ _ _ _ _ _ _ _ _ _ _ _ _ _ _ _ _ _ _ _ _ _ _ _ _ _] -> _
      tunnel: [_ _ _ "Adjust Scale\nto Mean" _ _ _ _ _ _ _ _ _ _ _ _ _ _ _ _ _ _ _ _ _ _ _ _ _ _ _ _ _ _ _ _ _ _ _ _ _ _ _ _ _ _ _ _ _ _ _ _ _ "Set SP to Reading" _ _] -> _
      tunnel: [_ _ _ _ _ _ _ _ _ "Round T2 X" _ "Delayed Interlace Start" _ _ _ _ _ _ _ _ _ _ _ _ _ _ _ _ _ _ _ _ _ _ _ _ _ _ _ _ _ _ _ _ _ _ _ _ _ _ _ _ _ _ _ _] -> _
      event "AI Count (ticks)", "Sets to FIFO (Traps)", "Save ave N", "FPGA Ave.", "# Samples/channel", "N sets to save": Value Change {
        # "So that if 'Save ave N' is updated, the AOD scanning code updates too."
        n1170 = event-data() -> ()  [unwired: 6 out]
        n1171 = local read "AI Count (ticks)"() -> (w4500:u32)
        n1172 = Boolean To (0,1)(Boolean="Sets to FIFO (Traps)") -> (0, 1=w4510:cluster{"Set 1":i16, "Set 2":i16, "Set 3":i16})
        n1173 = xnode "Read/Write Control"("FPGA VI Reference In"=w4520, "error in"=w4518, "ai count"=w4500, "AI1 Sets to FIFO"="Sets to FIFO (Traps)", "N of AI1 Int Acq Sets"="N Acq Sets (Traps + Fl.)") -> ("error out"=w4519:errorcluster)  [unwired: 1 out]
        n1174 = Cluster To Array(cluster=w4510) -> (array=w4509:i16[])
        n1175 = To Unsigned Long Integer(number=w4509) -> (unsigned 32bit integer=w4489:u32[])
        n1176 = local read "Scan steps (AOD)"() -> (w4511:u64)
        n1177 = Multiply(x=w4500, y="N Acq Sets (Traps + Fl.)") -> (x*y=w4498:u32)
        n1178 = Divide(x=40000000.0, y=w4500) -> (x/y=w4492:dbl)
        "AI rate (Hz)" <- w4492
        "Ave. Rate (Hz)" <- w4492
        n1179 = Add Array Elements(numeric array=w4489) -> (sum=w4501:u32)
        "Trap Sets" <- w4501
        n1180 = Reciprocal(x=w4492) -> (1/x=→"Ave. Period (s)":dbl)
        n1181 = property on="Scan steps (AOD)" class="DigNum (strict)"("Val(Sgnl)"=w4511) -> ()  [unwired: 2 in, 2 out]
        n1182 = Divide(x=w4492, y="N Acq Sets (Traps + Fl.)") -> (x/y=w4515:dbl)
        "Data Rate (Hz)" <- w4515
        n1183 = Reciprocal(x=w4515) -> (1/x=→"Data Period (s)":dbl)
        n1184 = local read "Save ave N"() -> (w4514:dbl)
        n1185 = Divide(x=w4515, y=w4514) -> (x/y=w4513:dbl)
        "Save Data Rate (Hz)" <- w4513
        n1186 = Reciprocal(x=w4513) -> (1/x=→"Save Data Period (s)":dbl)
        n1187 = Multiply(x=w4498, y="# Samples/trap") -> (x*y=w4496:u32)
        "Counts/DMA" <- w4496
        n1188 = property on="Trap Disp. Downsample" class="DigNum (strict)"("Maximum"="# Samples/trap") -> ()  [unwired: 2 in, 2 out]
        n1189 = Multiply(x=w4501, y="# Samples/trap") -> (x*y=w4490:u32)
        "# Samples/channel" <- w4490
        n1190 = Multiply(x=w4490, y=u32 8) -> (x*y=→"Trap AI Elements/DMA read":u32)
        n1191 = local read "APD Int. Count"() -> (w4497:u32)
        n1192 = Multiply(x=w4490, y=u32 3) -> (x*y=→"Trap Pos Elements/DMA read":u32)
        n1193 = Divide(x=w4496, y=w4497) -> (x/y=w4487:dbl)
        "APD Samples/FIFO Acq." <- w4487
        n1194 = Divide(x=w4496, y=40000000.0) -> (x/y=w4494:dbl)
        "DMA Update Period (s)" <- w4494
        n1195 = Multiply(x=2.0, y=w4487) -> (x*y=→"APD Elements/DMA read":dbl)
        n1196 = property on="APD Disp. Downsample" class="DigNum (strict)"("Maximum"=w4487) -> ()  [unwired: 2 in, 2 out]
        n1197 = local read "N sets to save"() -> (w4507:u32)
        n1198 = Multiply(x=w4494, y=w4507) -> (x*y=→"Total Time (s)":dbl)
        "FPGA Averaging" <- FALSE ("FPGA Averaging")
      }
      event "Rescale on Mean": Value Change {
        n1199 = event-data() -> ()  [unwired: 7 out]
        n1200 = And(x=FALSE, y="Rescale on Mean") -> (x .and. y?=w4607:bool)
        n1201 = local write "Rescale on Mean"(w4607) -> ()
        n1202 = local read "Bead Mean (nm)"() -> (w4612:dbl)
        n1203 = Add(x="Amplitude (nm)", y=w4612) -> (x+y=w4610:dbl)
        n1204 = Subtract(x=w4612, y="Amplitude (nm)") -> (x-y=w4609:dbl)
        n1205 = property on="Bead Separation" class="WFChart (strict)"("YScale.Minimum"=w4609) -> ()  [unwired: 2 in, 2 out]
        n1206 = property on="Bead Separation" class="WFChart (strict)"("YScale.Maximum"=w4610) -> ()  [unwired: 2 in, 2 out]
      }
      event "Detector Type": Value Change {
        n1207 = event-data() -> ()  [unwired: 7 out]
        n1208 = local read "AI labels"() -> (w4613:string[])
        n1209 = property on="High Res. Display" class="Ring (strict)"("Strings []"=w4613) -> ()  [unwired: 2 in, 2 out]
        n1210 = Build Array (concatenate)(w4613, "none") -> (w4614:string[])
        n1211 = property on="FFT 1 Choice 1" class="Ring (strict)"("Strings []"=w4614) -> ()  [unwired: 2 in, 2 out]
        n1212 = property on="FFT 1 Choice 2" class="Ring (strict)"("Strings []"=w4614) -> ()  [unwired: 2 in, 2 out]
        n1213 = property on="FFT 2 Choice 1" class="Ring (strict)"("Strings []"=w4614) -> ()  [unwired: 2 in, 2 out]
        n1214 = property on="FFT 2 Choice 2" class="Ring (strict)"("Strings []"=w4614) -> ()  [unwired: 2 in, 2 out]
        n1215 = Bundle("APD 1", "APD 2") -> (w4617:cluster{string, string})  [unwired: 1 out]
        n1216 = Cluster To Array(cluster=w4617) -> (array=w4615:string[])
        n1217 = Build Array (concatenate)(w4615, w4614) -> (w4619:string[])
        n1218 = Array Size(array=w4619) -> (size(s)=w4620:i32)
        n1219 = property on="Signals to Plot" class="LstBox (strict)"("Item Names"=w4619) -> ()  [unwired: 2 in, 2 out]
        n1220 = property on="Signals to Plot" class="LstBox (strict)"("Number of Rows"=w4620) -> ()  [unwired: 2 in, 2 out]
        n1221 = property on="All Signals" class="WFChart (strict)"("LegNumRows"=w4620) -> ()  [unwired: 2 in, 2 out]
      }
      event "Adjust Scale\nto Mean": Value Change {
        n1222 = event-data() -> ()  [unwired: 7 out]
        n1223 = local read "APD 1 Rate (Hz)"() -> (w4629:dbl)
        n1224 = Multiply(x=1000.0, y="Above (kHz)") -> (x*y=w4627:dbl)
        n1225 = Multiply(x=1000.0, y="Below (kHz)") -> (x*y=w4625:dbl)
        n1226 = Add(x=w4627, y=w4629) -> (x+y=w4622:dbl)
        n1227 = Subtract(x=w4629, y=w4625) -> (x-y=w4623:dbl)
        n1228 = property on="APD Chart" class="WFChart (strict)"("YScale.Minimum"=w4623) -> ()  [unwired: 2 in, 2 out]
        n1229 = property on="APD Chart" class="WFChart (strict)"("YScale.Maximum"=w4622) -> ()  [unwired: 2 in, 2 out]
      }
      event "Phase adj. (AI1)", "+ phase (AI1)", "- phase (AI1)": Value Change {
        n1230 = event-data() -> ()  [unwired: 7 out]
        n1231 = Negate(x="Phase adj. (AI1)") -> (-x=w4639:i16)
        n1232 = Select(t=w4639, s="- phase (AI1)", f="Phase adj. (AI1)") -> (s? t:f=w4638:i16)
        n1233 = xnode "Read/Write Control"("FPGA VI Reference In"=w4642, "error in"=w4641, "Phase count adjustment"=w4638) -> ("FPGA VI Reference Out"=w4637:T19, "error out"=w4636:errorcluster)
        n1234 = Or(x="- phase (AI1)", y="+ phase (AI1)") -> (x .or. y?=w4633:bool)
        n1235 = xnode "Read/Write Control"("FPGA VI Reference In"=w4637, "error in"=w4636, "+ phase"=w4633) -> ("error out"=w4632:errorcluster)  [unwired: 1 out]
      }
      event "Signals to Plot": Double Click {
        w4720 = u32 9868950 ("Color Box")
        n1236 = event-data() -> ("Row"=w4722:i32)  [unwired: 9 out]
        n1237 = property on="All Signals" class="WFChart (strict)"("Active Plot"=w4722) -> (error out=w4733:errorcluster)  [unwired: 2 in, 1 out]
        n1238 = property on="All Signals" class="WFChart (strict)" props=["Plot", "Visible?", "Plot", "Plot Color"](error in=w4733) -> (error out=w4732:errorcluster, "Plot.Visible?"=w4731:bool)  [unwired: 1 in, 2 out]
        n1239 = Select(t=FALSE ("Plot.Visible"), s=w4731, f=TRUE ("Plot.Visible")) -> (s? t:f=w4726:bool)
        n1240 = property on="All Signals" class="WFChart (strict)"(error in=w4732, "Plot.Visible?"=w4726) -> (error out=w4728:errorcluster)  [unwired: 1 in, 1 out]
        n1241 = property on="All Signals" class="WFChart (strict)"(error in=w4728) -> (error out=w4723:errorcluster, "Plot.Plot Color"=w4727:u32)  [unwired: 1 in, 1 out]
        n1242 = property on="Signals to Plot" class="LstBox (strict)"(error in=w4723, "Active Row"=w4722) -> (error out=w4721:errorcluster)  [unwired: 1 in, 1 out]
        n1243 = Select(t=w4727, s=w4726, f=u32 0) -> (s? t:f=w4724:u32)
        n1244 = property on="Signals to Plot" class="LstBox (strict)"(error in=w4721, "CellFontColor"=w4724, "SelColor"=w4720, "CellBG"=w4720, "CellFontSize"=u32 20 ("Active Row:Cell Font:Size"), "CellFontBold"=TRUE ("Active Row:Cell Font:Bold")) -> ()  [unwired: 1 in, 2 out]
      }
      event "BD 1 Frequency 1 (MHz)", "BD 1 Frequency 2 (MHz)", "BD 1 Frequency 3 (MHz)", "BD 2 Frequency 1 (MHz)", "BD 2 Frequency 2 (MHz)", "BD 2 Frequency 3 (MHz)", "Trap Delta (MHz)": Value Change {
        # "anytime one of the frequencies is changed, write it to the RF board UNLESS Set 1 is being oscillated. The oscillation\nscript writes the frequencies to the RF board."